vi "CompleteLabView.vi"() -> ()   [LabVIEW 2022 SP3]
panel:
  out "Selected time":string
  in  "UYST":bool
  in  "HST":bool
  in  "AKST":bool
  in  "PST":bool
  in  "MST":bool
  in  "CST":bool
  in  "EST":bool
  in  "NZST":bool
  in  "AEDT":bool
  in  "PGT":bool
  in  "JST":bool
  in  "HKT":bool
  in  "THA":bool
  in  "BST":bool
  in  "PKT":bool
  in  "GST":bool
  in  "AST":bool
  in  "CAT":bool
  in  "CET":bool
  in  "UTC":bool
  in  "CVT":bool
  in  "ART":bool
  in  "AST":bool
  in  "Hawaii-Aleutian Time (HST)":bool
  in  "Alaska Standard Time (AKST)":bool
  in  "Pacific Zone Time (PT)":bool
  in  "Eastern Standard Time (EST)":bool
  in  "Central Standard Time (CST)":bool
  in  "Mountain Time (MST) 16":bool
  in  "New Zealand Standard Time":bool
  in  "Australian Eastern Time (AEDT)":bool
  in  "Papua New Guinea Time (PGT)":bool
  in  "Japan Standard Time":bool
  in  "Hong Kong Time (HKT)":bool
  in  "Thailand Standard Time (THA)":bool
  in  "Bangladesh Standard Time (BST)":bool
  in  "Pakistan Standard Time":bool
  in  "Gulf Standard Time (GST)":bool
  in  "Arabia Standard Time (AST)":bool
  in  "Central Africa Time (CAT)":bool
  in  "Central European Time (CET)":bool
  in  "Coordinated Universal Time (UTC)":bool
  in  "Cape Verde Time (CVT)":bool
  in  "Uruguay Summer Time":bool
  in  "Argentina Time":bool
  in  "Atlantic Standard Time (AST)":bool
  in  "stop":bool
  out "Current UTC Time":string
  # "Directions:\n Please kick on desired time zone. On-click the time will display, but when release show the base time."
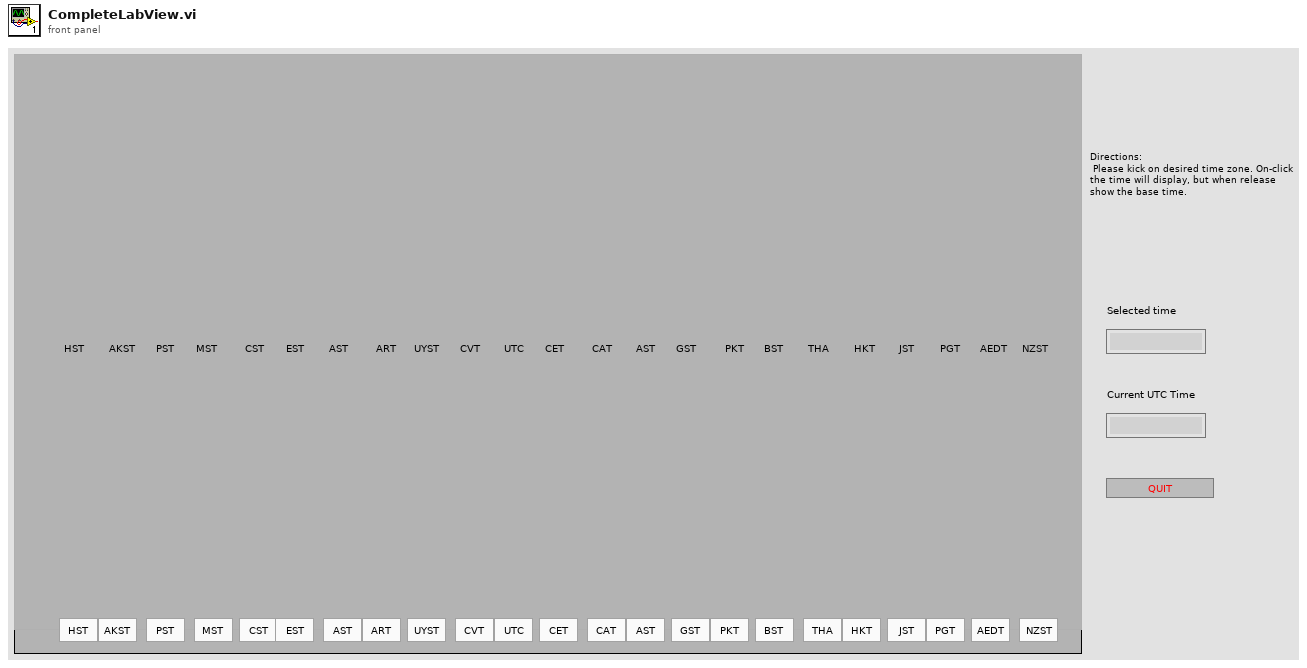
[diagram p1: front panel]
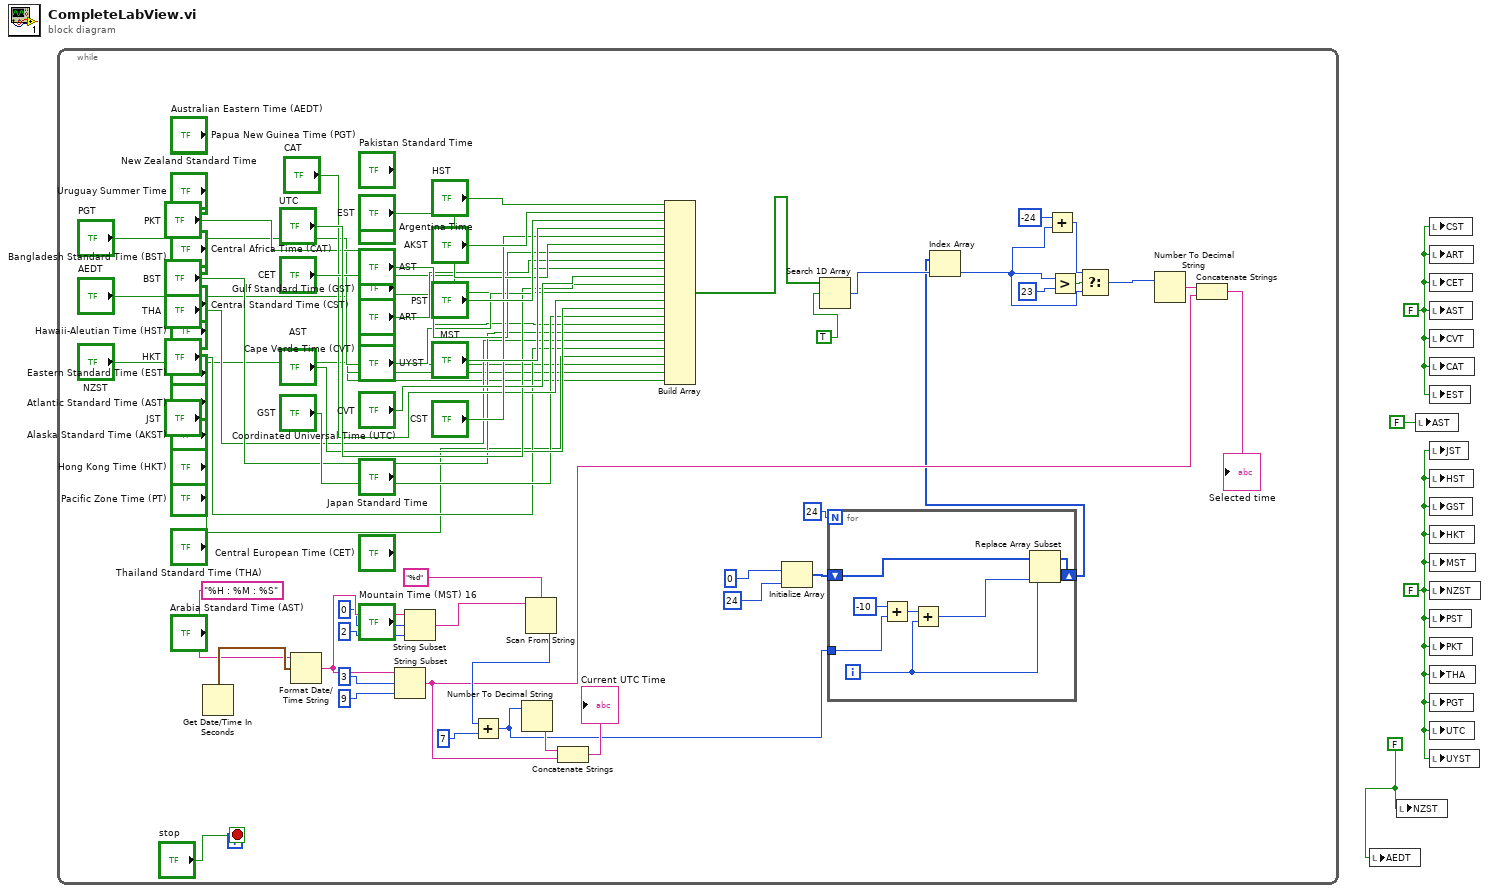
[diagram p0: block diagram]
diagram:
  w1 = FALSE
  w2 = FALSE
  w3 = FALSE
  n1 = while {
    stop <- "stop" stop-if-true
    n2 = Get Date/Time In Seconds() -> (seconds since 1Jan1904=w58:timestamp)
    n3 = Format Date/Time String(time format string (%c)="%H : %M : %S", seconds (now)=w58) -> (date/time string=w55:string)  [unwired: 1 in]
    n4 = String Subset(string=w55, offset (0)=3, length (rest)=9) -> (substring=w18:string)
    n5 = String Subset(string=w55, offset (0)=0, length (rest)=2) -> (substring=w57:string)
    n6 = Scan From String(format string="%d", input string=w57) -> (output 1=w56:i32)  [unwired: 3 in, 3 out]
    n7 = Add(x=w56, y=7) -> (x+y=w20:i32)
    n8 = Number To Decimal String(number=w20) -> (decimal integer string=w54:string)  [unwired: 1 in]
    n9 = Concatenate Strings(w54, w18) -> (→"Current UTC Time":string)
    n10 = Build Array("HST", "AKST", "PST", "MST", "CST", "EST", "AST", "ART", "UYST", "CVT", "UTC", "CET", "CAT", "AST", "GST", "PKT", "BST", "THA", "HKT", "JST", "PGT", "AEDT", "NZST") -> (w5:bool[])
    n11 = Initialize Array(0, 24) -> (w15:i32[])
    n12 = Search 1D Array(1D array=w5, element=TRUE) -> (index of element=w19:i32)  [unwired: 1 in]
    n13 = for {
      N: 24 -> [_]
      shift-right: [w61] -> w12
      shift-left: w15 -> [w63]
      tunnel: w20 -> [w65]
      i -> [w62]
      n14 = Add(x=-10, y=w65) -> (x+y=w64:i32)
      n15 = Add(x=w64, y=w62) -> (x+y=w60:i32)
      n16 = Replace Array Subset(array=w63, new element=w60, index=w62) -> (w61:i32[])
    }
    n17 = Index Array(array=w12, index=w19) -> (element=w9:i32)
    n18 = Add(x=-24, y=w9) -> (x+y=w8:i32)
    n19 = Greater?(x=w9, y=23) -> (0:w10:bool)
    n20 = Select(t=w8, s=w10, f=w9) -> (s? t:f=w7:i32)
    n21 = Number To Decimal String(number=w7) -> (decimal integer string=w17:string)  [unwired: 1 in]
    n22 = Concatenate Strings(w17, w18) -> (→"Selected time":string)
  }
  n23 = local write "AEDT"(w1) -> ()
  n24 = local write "NZST"(w1) -> ()
  n25 = local write "AST"(FALSE) -> ()
  n26 = local write "CST"(w3) -> ()
  n27 = local write "ART"(w3) -> ()
  n28 = local write "CET"(w3) -> ()
  n29 = local write "AST"(w3) -> ()
  n30 = local write "CVT"(w3) -> ()
  n31 = local write "CAT"(w3) -> ()
  n32 = local write "EST"(w3) -> ()
  n33 = local write "JST"(w2) -> ()
  n34 = local write "HST"(w2) -> ()
  n35 = local write "GST"(w2) -> ()
  n36 = local write "HKT"(w2) -> ()
  n37 = local write "MST"(w2) -> ()
  n38 = local write "NZST"(w2) -> ()
  n39 = local write "PST"(w2) -> ()
  n40 = local write "PKT"(w2) -> ()
  n41 = local write "THA"(w2) -> ()
  n42 = local write "PGT"(w2) -> ()
  n43 = local write "UTC"(w2) -> ()
  n44 = local write "UYST"(w2) -> ()
